vi "HFRR ADV v041.vi"() -> ()   [LabVIEW 2025] (continued)
                n816 = local write "Sample Temperature Calibration"(enum32{"True", "Fail"}."Fail" ("Sample Temperature Calibration  2")) -> ()
              }
              frame True {
                n817 = local write "Sample Temperature Calibration"(enum32{"True", "Fail"}."True" ("Sample Temperature Calibration  2")) -> ()
                n818 = property on="Accept & Save Air Temperature step 4" class="Bool (strict)"("DisabledEnum"=T19."Enabled" ("Disabled")) -> ()  [unwired: 2 in, 2 out]
              }
            }
          }
          frame #8 {
            # "CAL;END"
          }
          frame #9 {
            n819 = local write "Tab Control 4"(T12."Air Step 4" ("Tab Control 4")) -> ()
          }
        }
      }
      event "Back Stroke step main temperature": Value Change {
        n820 = event-data() -> ()  [unwired: 1 in, 6 out]
        n821 = stacked-sequence {
          frame #0 {
            n822 = Wait (ms)(milliseconds to wait=u32 1000) -> ()  [unwired: 1 out]
          }
          frame #1 {
            # "CAL;END"
            n823 = local write "Due Write"("CAL;END" ("Command")) -> ()
          }
          frame #2 {
            n824 = Wait (ms)(milliseconds to wait=u32 1000) -> ()  [unwired: 1 out]
          }
          frame #3 {
            # "CAL;END"
            n825 = local write "Due Write"("CAL;END" ("Command")) -> ()
          }
          frame #4 {
            n826 = local write "Temperature Selection"(T13."Default" ("Temperature Selection")) -> ()
            n827 = local write "Calibration Selection"(T8."Default" ("Calibration Selection")) -> ()
            n828 = local write "Main Calibration Tab"(T7."Main" ("Main Calibration Tab")) -> ()
            n829 = local write "Tab Control 4"(T12."Main" ("Tab Control 4")) -> ()
          }
        }
      }
      event "TEMPERATURE STEP  Back 4", "TEMPERATURE STEP 1 Back 3", "TEMPERATURE STEP  Back 3", "TEMPERATURE STEP 1 Back 2", "Back Air TEMPERATURE Step 4", "Back SAMPLE TEMPERATURE Step 4": Value Change {
        # "Back Stroke step main temperature"
        n830 = event-data() -> ()  [unwired: 1 in, 6 out]
        n831 = stacked-sequence {
          frame #0 {
            n832 = Wait (ms)(milliseconds to wait=u32 1000) -> ()  [unwired: 1 out]
          }
          frame #1 {
            # "CAL;END"
            n833 = local write "Due Write"("CAL;END" ("Command")) -> ()
          }
          frame #2 {
            n834 = Wait (ms)(milliseconds to wait=u32 1000) -> ()  [unwired: 1 out]
          }
          frame #3 {
            # "CAL;END"
            n835 = local write "Due Write"("CAL;END" ("Command")) -> ()
          }
          frame #4 {
            # "TEMPERATURE STEP  Back 4"
            n836 = local write "Main Calibration Tab"(T7."Temperature" ("Main Calibration Tab")) -> ()
            n837 = local write "Temperature Selection"(T13."Default" ("Temperature Selection")) -> ()
            n838 = local write "Tab Control 4"(T12."Main" ("Tab Control 4")) -> ()
            n839 = local write "Calibration Selection"(T8."Default" ("Calibration Selection")) -> ()
          }
        }
      }
      event "FF BACK", "FF BACK 2", "FF BACK 3", "FF BACK 4", "FF BACK 5", "FF BACK 6": Value Change {
        n840 = event-data() -> ()  [unwired: 1 in, 6 out]
        n841 = stacked-sequence {
          frame #0 {
            n842 = Wait (ms)(milliseconds to wait=u32 1500) -> ()  [unwired: 1 out]
          }
          frame #1 {
            n843 = local write "Due Write"("VC;0") -> ()
          }
          frame #2 {
            n844 = Wait (ms)(milliseconds to wait=u32 1500) -> ()  [unwired: 1 out]
          }
          frame #3 {
            n845 = local write "Due Write"("VC;0") -> ()
          }
          frame #4 {
            w875 = FALSE
            n846 = local write "FF BACK 2"(w875) -> ()
            n847 = local write "FF BACK 3"(w875) -> ()
            n848 = local write "FF BACK 4"(w875) -> ()
            n849 = local write "FF BACK 5"(w875) -> ()
            n850 = local write "FF BACK 6"(w875) -> ()
            n851 = local write "FF BACK"(w875) -> ()
          }
          frame #5 {
            n852 = local write "Temperature Selection"(T13."Default" ("Temperature Selection")) -> ()
            n853 = local write "Calibration Selection"(T8."Default" ("Calibration Selection")) -> ()
            n854 = local write "Friction Force Tab"(T25."Page 1" ("Friction Force Tab")) -> ()
            n855 = local write "Main Calibration Tab"(T7."Main" ("Main Calibration Tab")) -> ()
          }
        }
      }
      event "FF CONTINUE": Value Change {
        n856 = event-data() -> ()  [unwired: 1 in, 6 out]
        n857 = local write "FF CONTINUE"(FALSE ("FF CONTINUE")) -> ()
        n858 = local write "Friction Force Tab"(T25."Page 2" ("Friction Force Tab")) -> ()
      }
      event "FF CONTINUE 2": Value Change {
        n859 = event-data() -> ()  [unwired: 1 in, 6 out]
        n860 = local write "FF CONTINUE 2"(FALSE ("FF CONTINUE")) -> ()
        n861 = local write "Friction Force Tab"(T25."Page 3" ("Friction Force Tab")) -> ()
      }
      event "FF CONTINUE 3": Value Change {
        n862 = event-data() -> ()  [unwired: 1 in, 6 out]
        n863 = local write "FF CONTINUE 3"(FALSE ("FF CONTINUE")) -> ()
        n864 = local write "Friction Force Tab"(T25."Page 4" ("Friction Force Tab")) -> ()
      }
      event "FF CONTINUE 4": Value Change {
        n865 = event-data() -> ()  [unwired: 1 in, 6 out]
        n866 = local write "FF CONTINUE 4"(FALSE ("FF CONTINUE")) -> ()
        n867 = local write "Friction Force Tab"(T25."Page 5" ("Friction Force Tab")) -> ()
      }
      event "FF CONTINUE 5": Value Change {
        n868 = event-data() -> ()  [unwired: 1 in, 6 out]
        n869 = local write "FF CONTINUE 5"(FALSE ("FF CONTINUE")) -> ()
        n870 = local write "Friction Force Tab"(T25."Page 6" ("Friction Force Tab")) -> ()
      }
      event "Stroke Report Button": Value Change {
        n871 = event-data() -> ()  [unwired: 1 in, 6 out]
        n872 = local read "Point 5 - 1.0 mm"() -> (w891:bool)
        n873 = case shown="False" w891 {
          tunnel: [0.8 1.0] -> w890
          frame False {
          }
          frame True {
          }
        }
        n874 = local read "Machine Serial Number"() -> (w894:string)
        n875 = local read "USERNAME"() -> (w892:string)
        n876 = local write "Stroke Report Button"(FALSE ("Stroke Report Button")) -> ()
        n877 = call "Stroke Calibration Report.vi"("measured_value"=w890, "operator_name"=w892, "Instrument_serial Number"=w894) -> ()  [unwired: 7 in, 2 out]
      }
      event "Sample Report Button": Value Change {
        n878 = event-data() -> ()  [unwired: 1 in, 6 out]
        n879 = local read "Machine Serial Number"() -> (w900:string)
        n880 = local read "Sample 0deg temp"() -> (w897:dbl)
        n881 = local read "Sample 60deg temp"() -> (w898:dbl)
        n882 = local read "USERNAME"() -> (w899:string)
        n883 = call "Temperature Calibration Report.vi"("measured_60"=w898, "measured_zero"=w897, "operator_name"=w899, "Instrument_serial Number"=w900) -> ()  [unwired: 6 in, 2 out]
        n884 = local write "Sample Report Button"(FALSE ("Sample Report Button")) -> ()
      }
      event "Air Temperature Report Button": Value Change {
        n885 = event-data() -> ()  [unwired: 1 in, 6 out]
        n886 = local read "Machine Serial Number"() -> (w906:string)
        n887 = local read "Air 0deg temp"() -> (w903:dbl)
        n888 = local read "Air 60deg temp"() -> (w904:dbl)
        n889 = local read "USERNAME"() -> (w905:string)
        n890 = call "Air Temperature Calibration Report.vi"("measured_60"=w904, "measured_zero"=w903, "operator_name"=w905, "Instrument_serial Number"=w906) -> ()  [unwired: 6 in, 2 out]
        n891 = local write "Air Temperature Report Button"(FALSE ("Sample Report Button")) -> ()
      }
      event "Quit": Value Change {
        n892 = event-data() -> ()  [unwired: 1 in, 6 out]
      }
    }
    n893 = Wait (ms)(milliseconds to wait=u32 100) -> ()  [unwired: 1 out]
  }
  n894 = while {
    shift-right: [w909] -> _
    shift-left: "Enum - Selector" -> [w910]
    stop <- w911 stop-if-true
    # "Auto Start Logic Loop"
    n895 = case shown="\"close\"" w910 {
      tunnel: [w914 w920 w947 w979 w1009 Auto_Start_enum."Exit" ("Enum - Selector") Auto_Start_enum."Init" ("Enum - Selector")] -> w909
      frame "Init", Default {
        n896 = local read "Auto Start Test"() -> (w913:bool)
        n897 = Select(t=Auto_Start_enum."Humidity & Temperature On" ("Enum - Selector"), s=w913, f=Auto_Start_enum."Init") -> (s? t:f=w914:T15)
      }
      frame "Humidity & Temperature On" {
        n898 = stacked-sequence {
          tunnel: [_ _ _ _ _ _ Auto_Start_enum."Reach point" ("Enum - Selector")] -> w917
          frame #0 {
            w922 = T19."Disabled and Grayed Out" ("Disabled")
            w923 = TRUE ("Heater Button")
            n899 = property on="Humidity" class="Bool (strict)"("DisabledEnum"=w922) -> ()  [unwired: 2 in, 2 out]
            n900 = property on="Heater Button" class="Bool (strict)"("DisabledEnum"=w922) -> ()  [unwired: 2 in, 2 out]
            n901 = local write "Heater Button"(w923) -> ()
            n902 = local write "Humidity"(w923) -> ()
            n903 = property on="Heater Button" class="Bool (strict)"("Val(Sgnl)"=TRUE ("Value (Signaling)")) -> ()  [unwired: 2 in, 2 out]
          }
          frame #1 {
            n904 = Wait (ms)(milliseconds to wait=u32 3000) -> ()  [unwired: 1 out]
          }
          frame #2 {
            n905 = local read "Set Temp"() -> (w929:dbl)
            n906 = Number To Fractional String(number=w929, precision (6)=i16 2) -> (F-format string=w926:string)  [unwired: 2 in]
            n907 = Concatenate Strings("ST;" ("Command"), w926) -> (w927:string)
            n908 = local write "Due Write"(w927) -> ()
          }
          frame #3 {
            n909 = Wait (ms)(milliseconds to wait=u32 1500) -> ()  [unwired: 1 out]
          }
          frame #4 {
            (unwired) i16 2 ("precision (6)")
            n910 = local read "WriteHumidity"() -> (w931:string[])
            n911 = local read "Set Rh"() -> (w934:dbl)
            n912 = Number To Fractional String(number=w934) -> (F-format string=w935:string)  [unwired: 3 in]
            n913 = Concatenate Strings("M;" ("new element/subarray"), w935) -> (w936:string)
            n914 = Insert Into Array(array=w931, new element=w936) -> (w932:string[])  [unwired: 1 in]
            n915 = local write "WriteHumidity"(w932) -> ()
            n916 = local write "Due Write"("HE;1" ("Command")) -> ()
          }
          frame #5 {
            n917 = Wait (ms)(milliseconds to wait=u32 1500) -> ()  [unwired: 1 out]
          }
          frame #6 {
            w939 = TRUE ("Reach point temp")
            n918 = local write "Reach point Humidity"(w939) -> ()
            n919 = local write "Reach point temp"(w939) -> ()
          }
        }
        n920 = local read "Auto Start Test"() -> (w919:bool)
        n921 = Not(x=w919) -> (.not. x?=w918:bool)
        n922 = Select(t=Auto_Start_enum."close", s=w918, f=w917) -> (s? t:f=w920:T15)
      }
      frame "Reach point" {
        w948 = TRUE ("PAUSE")
        w956 = 1.0 ("y")
        w959 = 1.0 ("y")
        n923 = local read "Set Temp"() -> (w941:dbl)
        n924 = local read "Set Humidity:"() -> (w955:dbl)
        n925 = local read "Humidity ( %RH )"() -> (w960:dbl)
        n926 = Add(x=w941, y=w959) -> (x+y=w958:dbl)
        n927 = Subtract(x=w941, y=w959) -> (x-y=w957:dbl)
        n928 = Add(x=w955, y=w956) -> (x+y=w954:dbl)
        n929 = Subtract(x=w955, y=w956) -> (x-y=w953:dbl)
        n930 = local read "TEMP"() -> (w961:dbl)
        n931 = In Range and Coerce(upper limit=w954, x=w960, lower limit=w953) -> (In Range?=w942:bool)  [unwired: 1 out]
        n932 = In Range and Coerce(upper limit=w958, x=w961, lower limit=w957) -> (In Range?=w943:bool)  [unwired: 1 out]
        n933 = case shown="True" w942 {
          frame False {
          }
          frame True {
            n934 = case shown="True" "Reach point Humidity" {
              selector: "Reach point Humidity" -> [_ w967]
              frame False {
              }
              frame True {
                n935 = local read "EVENT LOG"() -> (w964:string)
                n936 = Not(x=w967) -> (.not. x?=w966:bool)
                n937 = local write "Reach point Humidity"(w966) -> ()
                n938 = call "Event Log.vi"("Content"="Target Humidity reached", "EVENT LOG"=w964) -> ("EVENT LOG"=w965:string)  [unwired: 8 in, 1 out]
                n939 = local write "EVENT LOG"(w965) -> ()
              }
            }
          }
        }
        n940 = case shown="True" w943 {
          frame False {
          }
          frame True {
            n941 = case shown="True" "Reach point temp" {
              selector: "Reach point temp" -> [_ w973]
              frame False {
              }
              frame True {
                n942 = local read "EVENT LOG"() -> (w970:string)
                n943 = Not(x=w973) -> (.not. x?=w972:bool)
                n944 = local write "Reach point temp"(w972) -> ()
                n945 = call "Event Log.vi"("Content"="Target Temperature reached", "EVENT LOG"=w970) -> ("EVENT LOG"=w971:string)  [unwired: 8 in, 1 out]
                n946 = local write "EVENT LOG"(w971) -> ()
              }
            }
          }
        }
        n947 = local read "Auto Start Test"() -> (w946:bool)
        n948 = And(x=w943, y=w942) -> (x .and. y?=w952:bool)
        n949 = Select(t=Auto_Start_enum."Maintain Stage" ("Enum - Selector"), s=w952, f=Auto_Start_enum."Reach point" ("Enum - Selector")) -> (s? t:f=w949:T15)
        n950 = Not(x=w946) -> (.not. x?=w945:bool)
        n951 = Select(t=Auto_Start_enum."close", s=w945, f=w949) -> (s? t:f=w947:T15)
        n952 = call "ELAPSED TIMER VI.vi"("RESET"=w948, "PAUSE"=w948) -> ()  [unwired: 7 in, 3 out]
      }
      frame "Maintain Stage" {
        w988 = 2.0 ("y")
        w987 = 1.0 ("y")
        # "Humidity and  temperatures Set Point  have been reached"
        n953 = local read "Set Temp"() -> (w974:dbl)
        n954 = local read "Set Humidity:"() -> (w991:dbl)
        n955 = local read "Humidity ( %RH )"() -> (w994:dbl)
        n956 = Add(x=w974, y=w987) -> (x+y=w993:dbl)
        n957 = Subtract(x=w974, y=w987) -> (x-y=w992:dbl)
        n958 = local read "TEMP"() -> (w995:dbl)
        n959 = Add(x=w991, y=w988) -> (x+y=w990:dbl)
        n960 = Subtract(x=w991, y=w988) -> (x-y=w989:dbl)
        n961 = In Range and Coerce(upper limit=w993, x=w995, lower limit=w992) -> (In Range?=w986:bool)  [unwired: 1 out]
        n962 = In Range and Coerce(upper limit=w990, x=w994, lower limit=w989) -> (In Range?=w985:bool)  [unwired: 1 out]
        n963 = And(x=w986, y=w985) -> (x .and. y?=w984:bool)
        n964 = Not(x=w984) -> (.not. x?=w983:bool)
        n965 = call "ELAPSED TIMER VI.vi"("TARGET"=60.0, "RESET"=w983, "PAUSE"=FALSE) -> ("ELAPSED INDICATION"=w980:bool)  [unwired: 6 in, 2 out]
        n966 = case shown="True" w980 {
          tunnel: w980 -> [_ w998]
          tunnel: [Auto_Start_enum."Maintain Stage" ("Enum - Selector") w997] -> w978
          frame False {
          }
          frame True {
            n967 = stacked-sequence {
              tunnel: w998 -> [_ _ _ _ _]
              tunnel: [_ _ _ _ Auto_Start_enum."Start Stage" ("Enum - Selector")] -> w997
              frame #0 {
                n968 = local read "EVENT LOG"() -> (w1000:string)
                n969 = call "Event Log.vi"("Content"="Humidity and temperature set point has stabilized.", "EVENT LOG"=w1000) -> ("EVENT LOG"=w1001:string)  [unwired: 8 in, 1 out]
                n970 = local write "EVENT LOG"(w1001) -> ()
              }
              frame #1 {
                n971 = Wait (ms)(milliseconds to wait=u32 100) -> ()  [unwired: 1 out]
              }
              frame #2 {
                n972 = local read "EVENT LOG"() -> (w1004:string)
                n973 = call "Event Log.vi"("Content"="Auto Test Started", "EVENT LOG"=w1004) -> ("EVENT LOG"=w1005:string)  [unwired: 8 in, 1 out]
                n974 = local write "EVENT LOG"(w1005) -> ()
              }
              frame #3 {
                w1006 = TRUE ("RUN")
                n975 = local write "RUN"(w1006) -> ()
                n976 = property on="Auto Start Temp" class="Bool (strict)"("Val(Sgnl)"=w1006) -> ()  [unwired: 2 in, 2 out]
                "Auto Start Temp" <- w1006
              }
              frame #4 {
              }
            }
          }
        }
        n977 = local read "Auto Start Test"() -> (w977:bool)
        n978 = Not(x=w977) -> (.not. x?=w976:bool)
        n979 = Select(t=Auto_Start_enum."close", s=w976, f=w978) -> (s? t:f=w979:T15)
      }
      frame "Start Stage" {
        w1008 = TRUE ("PAUSE")
        n980 = local read "Auto Start Test"() -> (w1013:bool)
        n981 = Not(x=w1013) -> (.not. x?=w1012:bool)
        n982 = Select(t=Auto_Start_enum."close" ("Enum - Selector"), s=w1012, f=Auto_Start_enum."Start Stage" ("Enum - Selector")) -> (s? t:f=w1009:T15)
        n983 = call "ELAPSED TIMER VI.vi"("RESET"=w1008, "PAUSE"=w1008) -> ()  [unwired: 7 in, 3 out]
      }
      frame "close" {
        w1016 = FALSE ("Heater Button")
        n984 = local write "RUN"(w1016) -> ()
        n985 = local write "Heater Button"(w1016) -> ()
        n986 = local write "Humidity"(w1016) -> ()
        n987 = local write "Auto Start Test"(w1016) -> ()
        n988 = property on="Heater Button" class="Bool (strict)"("Val(Sgnl)"=FALSE ("Value (Signaling)")) -> ()  [unwired: 2 in, 2 out]
        n989 = local write "Humidity 2"(TRUE ("Humidity")) -> ()
      }
      frame "Exit" {
      }
    }
    n990 = Wait (ms)(milliseconds to wait=u32 100) -> ()  [unwired: 1 out]
    n991 = local read "Quit"() -> (w911:bool)
  }
  n992 = property on="Service Password Log" class="Str"("Visible"=w23) -> ()  [unwired: 2 in, 2 out]
  n993 = property on="Password 3" class="Clust (strict)"("Visible"=w23) -> ()  [unwired: 2 in, 2 out]
  n994 = while {
    stop <- w1045 stop-if-true
    w1028 = errorcluster {"status"=FALSE, "code"=0, "source"=""} ("error in (no error) 3")
    # "this loop is for manual report generation"
    n995 = local read "Confirm Measrurement"() -> (w1027:bool)
    n996 = case shown="True" w1027 {
      selector: w1027 -> [_ w1135]
      tunnel: errorcluster {"status"=FALSE, "code"=0, "source"=""} ("error in (no error) 3") -> [_ w1136]
      tunnel: [_ w1134] -> _
      frame False {
      }
      frame True {
        n997 = stacked-sequence {
          tunnel: w1136 -> [_ w1169 _]
          tunnel: w1135 -> [_ _ w1276]
          tunnel: [_ w1157 _] -> w1134
          frame #0 {
            n998 = String To Path(string="C:\\LAB-IQ\\Image Calibrate v01.dcf") -> (path=w1139:path)
            n999 = Open/Create/Replace File ("Open File")(file path (use dialog)=w1139) -> (refnum out=w1140:refnum<file>)  [unwired: 5 in, 2 out]
            n1000 = for {
              N: 4 -> [_]
              tunnel: w1140 -> [w1146]
              i -> [w1142]
              n1001 = Read from Text File ("Read File")(file (use dialog)=w1146) -> (text=w1147:string)  [unwired: 3 in, 3 out]
              n1002 = String Subset(string=w1147, offset (0)=6, length (rest)=10 ("length (rest)")) -> (substring=w1143:string)
              n1003 = Fract/Exp String To Number(string=w1143) -> (number=w1141:dbl)  [unwired: 3 in, 1 out]
              n1004 = case shown="3" w1142 {
                tunnel: w1141 -> [w1148 w1149 _ w1150 _]
                frame 0 {
                  n1005 = local write "5x Gain"(w1148) -> ()
                }
                frame 1 {
                  n1006 = local write "10x Gain"(w1149) -> ()
                }
                frame 2 {
                }
                frame 3 {
                  n1007 = local write "100x gain"(w1150) -> ()
                }
                frame 4, Default {
                }
              }
            }
          }
          frame #1 {
            n1008 = local read "TEST STANDARD"() -> (w1152:T3)
            n1009 = case shown="\"ISO 12156\"" w1152 {
              tunnel: ["ASTM D6079" "ISO 12156"] -> w1151
              frame "ASTM D6079", Default {
              }
              frame "ISO 12156" {
              }
            }
            n1010 = call "IMAGE ANALYSIS.vi"("Enum"=POST_ANALYSIS_ENUM."GET MEASUREMENTS", "error in"=w1169) -> ("error out"=w1176:errorcluster)  [unwired: 8 in, 1 out]
            n1011 = local read "Magnification :"() -> (w1162:string)
            n1012 = call "Stall Data Flow.vim"("value in"=w1176, "milliseconds to wait"=u32 1000) -> ("value out"=w1175:errorcluster)  [unwired: 1 out]
            n1013 = local read "Test File List :"() -> (w1173:string)
            n1014 = case shown="\"10x\"" w1162 {
              tunnel: [w1212 w1213] -> w1160
              frame "5x", Default {
                n1015 = local read "5x Gain"() -> (w1212:dbl)
              }
              frame "10x" {
                # "5x"
                n1016 = local read "10x Gain"() -> (w1213:dbl)
              }
            }
            n1017 = call "IMAGE ANALYSIS.vi"("Enum"=POST_ANALYSIS_ENUM."READ", "error in"=w1175) -> ("error out"=w1172:errorcluster, "data out"=w1163:string)  [unwired: 8 in]
            n1018 = Match Pattern(string=w1163, regular expression="\"type\": ") -> (after substring=w1167:string)  [unwired: 1 in, 3 out]
            n1019 = call "IMAGE PATH CREATION PY.vi"("error in (no error)"=w1172, "File Name :"=w1173) -> ("error out"=w1171:errorcluster, "File Path"=w1159:path, "File Path String:"=w1154:string)  [unwired: 7 in]
            n1020 = Match Pattern(string=w1167, regular expression=",") -> (before substring=w1153:string)  [unwired: 1 in, 3 out]
            n1021 = local read "Calibration Tab"() -> (w1156:enum32{"Measrument", "Calibrate"})
            n1022 = call "Stall Data Flow.vim"("value in"=w1171, "milliseconds to wait"=u32 250) -> ("value out"=w1155:errorcluster)  [unwired: 1 out]
            n1023 = Equal?(x=w1153, y="\"rectangle\"") -> (x = y?=w1164:bool)
            n1024 = case shown="False" w1164 {
              tunnel: w1163 -> [w1218 w1273]
              tunnel: w1160 -> [_ w1264]
              tunnel: cluster{"major":dbl, "minor":dbl, "average":dbl} {"major"=0.0, "minor"=0.0, "average"=0.0} -> [w1216 w1260]
              tunnel: [w1215 w1257] -> w1158
              tunnel: w1153 -> [w1217 _]
              tunnel: w1160 -> [w1214 _]
              frame False {
                n1025 = Equal?(x=w1217, y="\"line\"") -> (x = y?=w1219:bool)
                n1026 = case shown="True" w1219 {
                  tunnel: w1218 -> [_ w1234]
                  tunnel: w1216 -> [w1221 w1233]
                  tunnel: [w1221 w1231] -> w1215
                  tunnel: w1214 -> [_ w1230]
                  frame False {
                  }
                  frame True {
                    w1229 = 0.0 ("Major Axis")
                    n1027 = Match Pattern(string=w1234, regular expression="\"length_px\":") -> (after substring=w1232:string)  [unwired: 1 in, 3 out]
                    n1028 = property on="Major Axis" class="DigNum (strict)"("Caption.Text"="") -> ()  [unwired: 2 in, 2 out]
                    n1029 = property on="Minor Axis" class="DigNum (strict)"("Caption.Text"="") -> ()  [unwired: 2 in, 2 out]
                    n1030 = property on="Average" class="DigNum (strict)"("Caption.Text"="Line") -> ()  [unwired: 2 in, 2 out]
                    n1031 = Fract/Exp String To Number(string=w1232, default (0 dbl)=0.0 ("default (0 DBL)")) -> (number=w1228:dbl)  [unwired: 2 in, 1 out]
                    "Pixel Value" <- w1228
                    n1032 = Multiply(x=w1228, y=w1230) -> (x*y=w1241:dbl)
                    n1033 = Multiply(x=w1241, y=1000.0) -> (x*y=w1224:dbl)
                    n1034 = Divide(x=w1224, y=1000.0) -> (x/y=w1227:dbl)
                    n1035 = local write "Measurment (mm)"(w1227) -> ()
                    n1036 = Bundle By Name(cluster=w1233, "average"=w1224) -> (w1231:cluster{"major":dbl, "minor":dbl, "average":dbl})
                    n1037 = Number To Fractional String(number=w1224, precision (6)=i16 1) -> (F-format string=w1223:string)  [unwired: 2 in]
                    n1038 = local write "Minor Axis"(w1229) -> ()
                    n1039 = local write "Major Axis"(w1229) -> ()
                    n1040 = Fract/Exp String To Number(string=w1223) -> (number=w1222:dbl)  [unwired: 3 in, 1 out]
                    n1041 = local write "Average"(w1222) -> ()
                  }
                }
              }
              frame True {
                w1261 = 1000.0 ("y")
                w1267 = 0.0 ("default (0 DBL)")
                n1042 = Match Pattern(string=w1273, regular expression=" \"width_px\":") -> (after substring=w1271:string)  [unwired: 1 in, 3 out]
                n1043 = Match Pattern(string=w1271, regular expression="\"height_px\":") -> (before substring=w1269:string, after substring=w1268:string)  [unwired: 1 in, 2 out]
                n1044 = Fract/Exp String To Number(string=w1269, default (0 dbl)=w1267) -> (number=w1266:dbl)  [unwired: 2 in, 1 out]
                n1045 = Fract/Exp String To Number(string=w1268, default (0 dbl)=w1267) -> (number=w1265:dbl)  [unwired: 2 in, 1 out]
                n1046 = Multiply(x=w1266, y=w1264) -> (x*y=w1263:dbl)
                n1047 = Multiply(x=w1265, y=w1264) -> (x*y=w1262:dbl)
                n1048 = Multiply(x=w1263, y=w1261) -> (x*y=w1247:dbl)
                n1049 = Multiply(x=w1262, y=w1261) -> (x*y=w1245:dbl)
                n1050 = Add(x=w1247, y=w1245) -> (x+y=w1259:dbl)
                n1051 = property on="Major Axis" class="DigNum (strict)"("Caption.Text"="Major Axis") -> ()  [unwired: 2 in, 2 out]
                n1052 = property on="Minor Axis" class="DigNum (strict)"("Caption.Text"="Minor Axis") -> ()  [unwired: 2 in, 2 out]
                n1053 = property on="Average" class="DigNum (strict)"("Caption.Text"="Average") -> ()  [unwired: 2 in, 2 out]
                n1054 = Divide(x=w1259, y=2.0) -> (x/y=w1243:dbl)
                n1055 = Bundle By Name(cluster=w1260, "major"=w1247, "minor"=w1245, "average"=w1243) -> (w1257:cluster{"major":dbl, "minor":dbl, "average":dbl})
                n1056 = Number To Fractional String(number=w1245, precision (6)=i16 1) -> (F-format string=w1252:string)  [unwired: 2 in]
                n1057 = Number To Fractional String(number=w1243, precision (6)=i16 1) -> (F-format string=w1253:string)  [unwired: 2 in]
                n1058 = Number To Fractional String(number=w1247, precision (6)=i16 1) -> (F-format string=w1251:string)  [unwired: 2 in]
                n1059 = Fract/Exp String To Number(string=w1252) -> (number=w1244:dbl)  [unwired: 3 in, 1 out]
                n1060 = Fract/Exp String To Number(string=w1253) -> (number=w1242:dbl)  [unwired: 3 in, 1 out]
                n1061 = Fract/Exp String To Number(string=w1251) -> (number=w1246:dbl)  [unwired: 3 in, 1 out]
                n1062 = local write "Major Axis"(w1246) -> ()
                n1063 = local write "Average"(w1242) -> ()
                n1064 = local write "Minor Axis"(w1244) -> ()
              }
            }
            n1065 = case shown="\"Measrument\", Default" w1156 {
              tunnel: w1159 -> [w1186 _]
              tunnel: w1158 -> [w1185 _]
              tunnel: [w1182 w1211] -> w1157
              tunnel: w1155 -> [w1184 w1211]
              tunnel: w1154 -> [w1183 _]
              tunnel: w1151 -> [w1181 _]
              frame "Measrument", Default {
                n1066 = stacked-sequence {
                  tunnel: w1186 -> [w1204 _]
                  tunnel: w1185 -> [w1202 _]
                  tunnel: w1184 -> [w1200 _]
                  tunnel: w1183 -> [w1199 _]
                  tunnel: [w1194 _] -> w1182
                  tunnel: w1181 -> [w1187 _]
                  frame #0 {
                    n1067 = call "IMAGE ANALYSIS.vi"("Enum"=POST_ANALYSIS_ENUM."SAVE IMAGE", "error in"=w1200, "IMAGE FILE PATH"=w1199) -> ("error out"=w1198:errorcluster)  [unwired: 7 in, 1 out]
                    n1068 = call "Stall Data Flow.vim"("value in"=w1198, "milliseconds to wait"=u32 1000) -> ("value out"=w1189:errorcluster)  [unwired: 1 out]
                    n1069 = local read "Test File List :"() -> (w1206:string)
                    n1070 = call "IMAGE ANALYSIS.vi"("Enum"=POST_ANALYSIS_ENUM."MINIMIZE UI", "error in"=w1189) -> ("error out"=w1196:errorcluster)  [unwired: 8 in, 1 out]
                    n1071 = Bundle By Name(cluster=T27 {"File Name"="", "Test Method"="", "Operator"="", "Fuel Description"="", "Date and time"=""} ("Main Ref"), "Test Method"=w1187, "File Name"=w1206) -> (w1207:T27)
                    n1072 = call "Stall Data Flow.vim"("value in"=w1196, "milliseconds to wait"=u32 1500) -> ("value out"=w1191:errorcluster)  [unwired: 1 out]
                    n1073 = call "duf file read.vi"("error in (no error)"=w1191, "Main Ref"=w1207) -> ("error out"=w1205:errorcluster, "Main Ref 2"=w1203:T27)  [unwired: 8 in]
                    n1074 = call "DETECTION REPORT for manual.vi"("error in (no error)"=w1205, "return value 3"=w1202, "Image File Path"=w1204, "Main Ref"=w1203) -> ("error out"=w1201:errorcluster)  [unwired: 7 in]
                    n1075 = call <vilib>:"Clear Errors.vi"("error in (no error)"=w1201) -> ("error out"=w1192:errorcluster)  [unwired: 5 in, 1 out]
                    n1076 = call "IMAGE ANALYSIS.vi"("Enum"=POST_ANALYSIS_ENUM."MINIMIZE UI", "error in"=w1192) -> ("error out"=w1194:errorcluster)  [unwired: 8 in, 1 out]
                  }
                  frame #1 {
                    n1077 = local write "Main Tab"(T2."HOME" ("Main Tab")) -> ()
                    n1078 = local write "Main Dashboard Buttons"(T1."Home" ("Main Dashboard Buttons")) -> ()
                  }
                }
              }
              frame "Calibrate" {
              }
            }
          }
          frame #2 {
            n1079 = Not(x=w1276) -> (.not. x?=w1275:bool)
            n1080 = local write "Confirm Measrurement"(w1275) -> ()
            n1081 = local read "Calibration Tab"() -> (w1274:enum32{"Measrument", "Calibrate"})
            n1082 = case shown="\"Measrument\", Default" w1274 {
              frame "Measrument", Default {
                (unwired) T21."HOME" ("Main Tab")
                n1083 = local write "Main Tab"(T2."HOME" ("Main Tab")) -> ()
              }
              frame "Calibrate" {
              }
            }
          }
        }
      }
    }
    n1084 = local read "Humidity"() -> (w1019:bool)
    n1085 = local read "Save Change"() -> (w1024:bool)
    n1086 = local read "Calibrate"() -> (w1025:bool)
    n1087 = local read "Auto Start Test"() -> (w1020:bool)
    n1088 = case shown="True" w1025 {
      selector: w1025 -> [_ w1132]
      frame False {
      }
      frame True {
        n1089 = Not(x=w1132) -> (.not. x?=w1131:bool)
        n1090 = local write "Calibrate"(w1131) -> ()
        n1091 = local write "Calibration Tab"(enum32{"Measrument", "Calibrate"}."Calibrate" ("Calibration Tab")) -> ()
      }
    }
    n1092 = case shown="True" w1024 {
      selector: w1024 -> [_ w1076]
      frame False {
      }
      frame True {
        n1093 = stacked-sequence {
          tunnel: w1076 -> [_ _ _ _ w1130]
          frame #0 {
            n1094 = call "IMAGE ANALYSIS.vi"("Enum"=POST_ANALYSIS_ENUM."HIDE UI") -> ()  [unwired: 9 in, 2 out]
          }
          frame #1 {
            n1095 = local read "100x gain"() -> (w1078:dbl)
            n1096 = local read "10x Gain"() -> (w1079:dbl)
            n1097 = local read "5x Gain"() -> (w1080:dbl)
            n1098 = Number To Fractional String(number=w1079, width (-)=i16 4, precision (6)=i16 7) -> (F-format string=w1101:string)  [unwired: 1 in]
            n1099 = Number To Fractional String(number=0.0, width (-)=i16 4, precision (6)=i16 7) -> (F-format string=w1096:string)  [unwired: 1 in]
            n1100 = Number To Fractional String(number=w1078, width (-)=i16 4, precision (6)=i16 7) -> (F-format string=w1084:string)  [unwired: 1 in]
            n1101 = Number To Fractional String(number=w1080, width (-)=i16 10 ("precision (6)"), precision (6)=i16 7) -> (F-format string=w1110:string)  [unwired: 1 in]
            n1102 = Concatenate Strings("[CH1]" ("string"), w1110, " - 5x Gain" ("string"), "\r") -> (w1100:string)
            n1103 = Concatenate Strings("[CH2]" ("string"), w1101, " - 10x Gain" ("string"), "\r") -> (w1099:string)
            n1104 = Concatenate Strings("[CH3]" ("string"), w1096, " - 20x Gain" ("string"), "\r") -> (w1090:string)
            n1105 = Concatenate Strings("[CH4]" ("string"), w1084, " - 100x Gain" ("string"), "\r") -> (w1083:string)
            n1106 = String To Path(string="C:\\LAB-IQ\\Image Calibrate v01.dcf") -> (path=w1113:path)
            n1107 = Concatenate Strings(w1100, w1099, w1090, w1083) -> (w1098:string)
            n1108 = call <vilib>:"Write Characters To File.vi"("append to file? (new file:F)"=FALSE, "character string"=w1098, "file path (dialog if empty)"=w1113) -> ()  [unwired: 2 in, 1 out]
          }
          frame #2 {
            n1109 = String To Path(string="C:\\LAB-IQ\\Image Calibrate v01.dcf") -> (path=w1116:path)
            n1110 = Open/Create/Replace File ("Open File")(file path (use dialog)=w1116) -> (refnum out=w1117:refnum<file>)  [unwired: 5 in, 2 out]
            n1111 = for {
              N: 4 -> [_]
              tunnel: w1117 -> [w1123]
              i -> [w1119]
              n1112 = Read from Text File ("Read File")(file (use dialog)=w1123) -> (text=w1124:string)  [unwired: 3 in, 3 out]
              n1113 = String Subset(string=w1124, offset (0)=6, length (rest)=10 ("length (rest)")) -> (substring=w1120:string)
              n1114 = Fract/Exp String To Number(string=w1120) -> (number=w1118:dbl)  [unwired: 3 in, 1 out]
              n1115 = case shown="3" w1119 {
                tunnel: w1118 -> [w1125 w1126 _ w1127 _]
                frame 0 {
                  n1116 = local write "5x Gain"(w1125) -> ()
                }
                frame 1 {
                  n1117 = local write "10x Gain"(w1126) -> ()
                }
                frame 2 {
                }
                frame 3 {
                  n1118 = local write "100x gain"(w1127) -> ()
                }
                frame 4, Default {
                }
              }
            }
          }
          frame #3 {
            n1119 = call "IMAGE ANALYSIS.vi"("Enum"=POST_ANALYSIS_ENUM."SHOW UI") -> ()  [unwired: 9 in, 2 out]
          }
          frame #4 {
            n1120 = Not(x=w1130) -> (.not. x?=w1129:bool)
            n1121 = local write "Save Change"(w1129) -> ()
          }
        }
      }
    }
    n1122 = case shown="False" w1020 {
      tunnel: w1019 -> [w1046 _]
      frame False {
        n1123 = case shown="True" w1046 {
          frame False {
          }
          frame True {
            n1124 = local read "Set Humidity:"() -> (w1050:dbl)
            n1125 = local read "Set Humidity:"() -> (w1053:dbl)
            n1126 = local read "Humidity ( %RH )"() -> (w1054:dbl)
            n1127 = Subtract(x=w1050, y=2.0) -> (x-y=w1048:dbl)
            n1128 = Add(x=w1053, y=2.0) -> (x+y=w1049:dbl)
            n1129 = In Range and Coerce(upper limit=w1049, x=w1054, lower limit=w1048) -> (In Range?=w1047:bool)  [unwired: 1 out]
            n1130 = case shown="True" w1047 {
              frame False {
              }
              frame True {
                n1131 = case shown="True" "Manual Humididty Reached" {
                  selector: "Manual Humididty Reached" -> [_ w1057]
                  frame False {
                  }
                  frame True {
                    n1132 = Not(x=w1057) -> (.not. x?=w1056:bool)
                    n1133 = local write "Manual Humididty Reached"(w1056) -> ()
                    n1134 = local read "EVENT LOG"() -> (w1059:string)
                    n1135 = call "Event Log.vi"("Content"="Target Humidity reached", "EVENT LOG"=w1059) -> ("EVENT LOG"=w1058:string)  [unwired: 8 in, 1 out]
                    n1136 = local write "EVENT LOG"(w1058) -> ()
                  }
                }
              }
            }
          }
        }
      }
      frame True {
        n1137 = local write "Manual Humididty Reached"(TRUE ("Manual Humididty Reached")) -> ()
      }
    }
    n1138 = local read "Cap Live Image"() -> (w1040:bool)
    n1139 = local read "SCAR MEASURMENT"() -> (w1043:enum32{"Auto Scar", "Manual Scar"})
    n1140 = Equal?(x=w1043, y=enum32{"Auto Scar", "Manual Scar"}."Manual Scar" ("SCAR MEASURMENT")) -> (x = y?=w1041:bool)
    n1141 = And(x=w1041, y=w1040) -> (x .and. y?=w1039:bool)
    n1142 = Wait (ms)(milliseconds to wait=u32 250) -> ()  [unwired: 1 out]
    n1143 = case shown="True" w1039 {
      selector: w1039 -> [_ w1362]
      frame False {
      }
      frame True {
        n1144 = stacked-sequence {
          tunnel: [_ _ _ w1381 _] -> _
          tunnel: w1362 -> [_ _ _ _ w1388]
          frame #0 {
            w1363 = 0.0
            n1145 = local write "Major Axis"(w1363) -> ()
            n1146 = local write "Minor Axis"(w1363) -> ()
            n1147 = local write "Average"(w1363) -> ()
          }
          frame #1 {
            n1148 = call "CAMERA LIVE FEED FGV.vi"("Enum - Menu"=CAMERA_LIVE_FEED_ENUM."CAMERA MINIMIZE") -> ()  [unwired: 9 in, 2 out]
          }
          frame #2 {
            n1149 = local read "Magnification len live scar"() -> (w1367:string)
            n1150 = case shown="\"10x\", Default" w1367 {
              tunnel: ["_10x" "_5x"] -> w1366
              frame "10x", Default {
              }
              frame "5x" {
              }
            }
            n1151 = local read "FILE 3"() -> (w1373:string)
            n1152 = call <vilib>:"Trim Whitespace.vi"("string"="C:\\LAB-IQ\\images\\") -> ("trimmed string"=w1375:string)  [unwired: 1 in]
            n1153 = String To Path(string=w1375) -> (path=w1374:path)
            n1154 = Concatenate Strings(w1373, w1366, ".png" ("string")) -> (w1372:string)
            n1155 = Build Path(base path=w1374, name or relative path=w1372) -> (appended path=w1371:path)
            n1156 = Path To String(path=w1371) -> (string=w1370:string)
            n1157 = call "CAMERA LIVE FEED FGV.vi"("Enum - Menu"=CAMERA_LIVE_FEED_ENUM."CAMERA SAVE", "Image Path"=w1370) -> ("error out"=w1368:errorcluster)  [unwired: 8 in, 1 out]
            n1158 = case shown="No Error" w1368 {
              frame No Error {
                n1159 = One Button Dialog(message="Image saved successfully") -> ()  [unwired: 1 in, 1 out]
              }
              frame Error {
              }
            }
          }
          frame #3 {
            n1160 = call "LIST FILE NAMES.vi"() -> ("error out"=w1383:errorcluster, "filenames"=w1380:string[])  [unwired: 10 in]
            n1161 = call "IMAGE ANALYSIS.vi"("Enum"=POST_ANALYSIS_ENUM."SHOW UI", "error in"=w1383) -> ("error out"=w1381:errorcluster)  [unwired: 8 in, 1 out]
            n1162 = property on="Test File List :" class="CmbBox"("Strings[]"=w1380) -> ()  [unwired: 2 in, 2 out]
          }
          frame #4 {
            (unwired) T26."Report" ("Main Dashboard Buttons")
            (unwired) T28."Report" ("Main Dashboard Buttons")
            n1163 = Not(x=w1388) -> (.not. x?=w1387:bool)
            n1164 = local write "Zoom Factore"(0.0 ("Zoom Factore")) -> ()
            n1165 = local write "Cap Live Image"(w1387) -> ()
            n1166 = local write "Main Tab"(T2."Adv Scar Report" ("Main Tab")) -> ()
            n1167 = property on="Cap Live Image" class="Bool (strict)"("BoolText.Text"="Capture Image" ("Boolean Text.Text")) -> ()  [unwired: 2 in, 2 out]
            n1168 = local write "Main Dashboard Buttons"(T1."Report" ("Main Dashboard Buttons")) -> ()
          }
        }
      }
    }
    n1169 = local read "change Gain"() -> (w1023:bool)
    n1170 = local read "Back Square"() -> (w1022:bool)
    n1171 = case shown="True" w1023 {
      selector: w1023 -> [_ w1067]
      frame False {
      }
      frame True {
        n1172 = stacked-sequence {
          tunnel: w1067 -> [_ w1075]
          frame #0 {
            n1173 = local read "Actual (µm)"() -> (w1071:dbl)
            n1174 = local read "Pixel Value"() -> (w1070:dbl)
            n1175 = local read "Magnification :"() -> (w1069:string)
            n1176 = Divide(x=w1071, y=w1070) -> (x/y=w1068:dbl)
            n1177 = case shown="\"10x\"" w1069 {
              tunnel: w1068 -> [w1072 w1073]
              frame "10x" {
                n1178 = local write "10x Gain"(w1072) -> ()
              }
              frame "5x", Default {
                n1179 = local write "5x Gain"(w1073) -> ()
              }
            }
          }
          frame #1 {
            n1180 = Not(x=w1075) -> (.not. x?=w1074:bool)
            n1181 = local write "change Gain"(w1074) -> ()
          }
        }
      }
    }
    n1182 = case shown="True" w1022 {
      selector: w1022 -> [_ w1065]
      frame False {
      }
      frame True {
        n1183 = Not(x=w1065) -> (.not. x?=w1064:bool)
        n1184 = local write "Back Square"(w1064) -> ()
        n1185 = local write "Calibration Tab"(enum32{"Measrument", "Calibrate"}."Measrument" ("Calibration Tab")) -> ()
      }
    }
    n1186 = local read "Rectangle Tool"() -> (w1034:bool)
    n1187 = local read "Clear ROI Tool"() -> (w1033:bool)
    n1188 = local read "Open Image"() -> (w1038:bool)
    n1189 = local read "line tool"() -> (w1035:bool)
    n1190 = local read "OUT"() -> (w1036:bool)
    n1191 = local read "In"() -> (w1037:bool)
    n1192 = case shown="True" w1038 {
      selector: w1038 -> [_ w1348]
      tunnel: [w1339 w1350] -> _
      tunnel: w1028 -> [w1339 w1349]
      frame False {
      }
      frame True {
        w1343 = "_5x" ("regular expression")
        n1193 = Not(x=w1348) -> (.not. x?=w1347:bool)
        n1194 = local write "Open Image"(w1347) -> ()
        n1195 = call "IMAGE ANALYSIS.vi"("Enum"=POST_ANALYSIS_ENUM."HIDE UI", "error in"=w1349) -> ("error out"=w1357:errorcluster)  [unwired: 8 in, 1 out]
        n1196 = call <vilib>:"Clear Errors.vi"("error in (no error)"=w1357) -> ("error out"=w1340:errorcluster)  [unwired: 5 in, 1 out]
        n1197 = call "File Dialog"("start path"=path "C:/LAB-IQ/images", "error in"=w1340) -> ("selected path"=w1342:path, "error out"=w1355:errorcluster)  [unwired: 10 in, 2 out]
        "Image path  2" <- w1342
        n1198 = call <vilib>:"Clear Errors.vi"("error in (no error)"=w1355) -> ("error out"=w1354:errorcluster)  [unwired: 5 in, 1 out]
        n1199 = call "IMAGE ANALYSIS.vi"("Enum"=POST_ANALYSIS_ENUM."OPEN FILE", "error in"=w1354, "File Path"=w1342) -> ("error out"=w1353:errorcluster)  [unwired: 7 in, 1 out]
        n1200 = call <vilib>:"Clear Errors.vi"("error in (no error)"=w1353) -> ("error out"=w1352:errorcluster)  [unwired: 5 in, 1 out]
        n1201 = call "IMAGE ANALYSIS.vi"("Enum"=POST_ANALYSIS_ENUM."SHOW UI", "error in"=w1352) -> ("error out"=w1350:errorcluster)  [unwired: 8 in, 1 out]
        n1202 = local write "Zoom Factore"(100.0 ("Zoom Factore")) -> ()
        n1203 = Strip Path(path=w1342) -> (name=w1345:string)  [unwired: 1 out]
        n1204 = Match Pattern(string=w1345, regular expression=w1343) -> (match substring=w1344:string)  [unwired: 1 in, 3 out]
        n1205 = Equal?(x=w1344, y=w1343) -> (x = y?=w1341:bool)
        n1206 = case shown="False" w1341 {
          frame False {
            n1207 = local write "Magnification :"("10x" ("Magnification :")) -> ()
          }
          frame True {
            n1208 = local write "Magnification :"("5x" ("Magnification :")) -> ()
          }
        }
      }
    }
    n1209 = case shown="True" w1036 {
      selector: w1036 -> [_ w1324]
      tunnel: w1028 -> [w1321 w1329]
      tunnel: [w1321 w1323] -> _
      frame False {
      }
      frame True {
        n1210 = Not(x=w1324) -> (.not. x?=w1322:bool)
        n1211 = local read "Zoom Factore"() -> (w1327:dbl)
        n1212 = local write "OUT"(w1322) -> ()
        n1213 = call "IMAGE ANALYSIS.vi"("Enum"=POST_ANALYSIS_ENUM."ZOOM OUT", "error in"=w1329) -> ("error out"=w1323:errorcluster)  [unwired: 8 in, 1 out]
        n1214 = Divide(x=w1327, y=1.2) -> (x/y=w1325:dbl)
        n1215 = local write "Zoom Factore"(w1325) -> ()
      }
    }
    n1216 = case shown="True" w1037 {
      selector: w1037 -> [_ w1333]
      tunnel: w1028 -> [w1330 w1338]
      tunnel: [w1330 w1331] -> _
      frame False {
      }
      frame True {
        n1217 = Not(x=w1333) -> (.not. x?=w1332:bool)
        n1218 = local read "Zoom Factore"() -> (w1336:dbl)
        n1219 = local write "In"(w1332) -> ()
        n1220 = call "IMAGE ANALYSIS.vi"("Enum"=POST_ANALYSIS_ENUM."ZOOM IN", "error in"=w1338) -> ("error out"=w1331:errorcluster)  [unwired: 8 in, 1 out]
        n1221 = Multiply(x=w1336, y=1.2) -> (x*y=w1334:dbl)
        n1222 = local write "Zoom Factore"(w1334) -> ()
      }
    }
    n1223 = case shown="True" w1033 {
      selector: w1033 -> [_ w1305]
      tunnel: w1028 -> [w1303 w1307]
      tunnel: [w1303 w1306] -> _
      frame False {
      }
      frame True {
        n1224 = Not(x=w1305) -> (.not. x?=w1304:bool)
        n1225 = local write "Clear ROI Tool"(w1304) -> ()
        n1226 = call "IMAGE ANALYSIS.vi"("Enum"=POST_ANALYSIS_ENUM."CLEAR ROI", "error in"=w1307) -> ("error out"=w1306:errorcluster)  [unwired: 8 in, 1 out]
      }
    }
    n1227 = case shown="True" w1035 {
      selector: w1035 -> [_ w1317]
      tunnel: w1028 -> [w1315 w1320]
      tunnel: [w1315 w1318] -> _
      frame False {
      }
      frame True {
        n1228 = Not(x=w1317) -> (.not. x?=w1316:bool)
        n1229 = local write "line tool"(w1316) -> ()
        n1230 = call "IMAGE ANALYSIS.vi"("Enum"=POST_ANALYSIS_ENUM."DRAW LINE", "error in"=w1320) -> ("error out"=w1318:errorcluster)  [unwired: 8 in, 1 out]
      }
    }
    n1231 = case shown="True" w1034 {
      selector: w1034 -> [_ w1311]
      tunnel: w1028 -> [w1309 w1313]
      tunnel: [w1309 w1312] -> _
      frame False {
      }
      frame True {
        n1232 = Not(x=w1311) -> (.not. x?=w1310:bool)
        n1233 = local write "Rectangle Tool"(w1310) -> ()
        n1234 = call "IMAGE ANALYSIS.vi"("Enum"=POST_ANALYSIS_ENUM."DRAW REC", "error in"=w1313) -> ("error out"=w1312:errorcluster)  [unwired: 8 in, 1 out]
      }
    }
    n1235 = local read "SCAR MEASURMENT"() -> (w1021:enum32{"Auto Scar", "Manual Scar"})
    n1236 = local read "Fit to Screen Tool"() -> (w1030:bool)
    n1237 = local read "Resize Tool"() -> (w1029:bool)
    n1238 = case shown="\"Manual Scar\", Default" w1021 {
      frame "Auto Scar" {
        n1239 = property on="Cap Live Image" class="Bool (strict)"("BoolText.Text"="Report" ("Boolean Text.Text")) -> ()  [unwired: 2 in, 2 out]
      }
      frame "Manual Scar", Default {
        n1240 = property on="Cap Live Image" class="Bool (strict)"("BoolText.Text"="Save Image" ("Boolean Text.Text")) -> ()  [unwired: 2 in, 2 out]
      }
    }
    n1241 = local read "ROI Color Tool"() -> (w1031:bool)
    n1242 = local read "Pan Tool"() -> (w1032:bool)
    n1243 = case shown="True" w1032 {
      selector: w1032 -> [_ w1299]
      tunnel: w1028 -> [w1297 w1301]
      tunnel: [w1297 w1300] -> _
      frame False {
      }
      frame True {
        n1244 = Not(x=w1299) -> (.not. x?=w1298:bool)
        n1245 = call "IMAGE ANALYSIS.vi"("Enum"=POST_ANALYSIS_ENUM."PAN", "error in"=w1301) -> ("error out"=w1300:errorcluster)  [unwired: 8 in, 1 out]
        n1246 = local write "Pan Tool"(w1298) -> ()
      }
    }
    n1247 = case shown="True" w1029 {
      selector: w1029 -> [_ w1283]
      tunnel: w1028 -> [w1278 w1280]
      tunnel: [w1278 w1279] -> _
      frame False {
      }
      frame True {
        n1248 = Not(x=w1283) -> (.not. x?=w1282:bool)
        n1249 = local write "Resize Tool"(w1282) -> ()
        n1250 = call "IMAGE ANALYSIS.vi"("Enum"=POST_ANALYSIS_ENUM."RESIZE MODE", "error in"=w1280) -> ("error out"=w1279:errorcluster)  [unwired: 8 in, 1 out]
      }
    }
    n1251 = case shown="True" w1030 {
      selector: w1030 -> [_ w1288]
      tunnel: [w1284 w1289] -> _
      tunnel: w1028 -> [w1284 w1287]
      frame False {
      }
      frame True {
        n1252 = Not(x=w1288) -> (.not. x?=w1286:bool)
        n1253 = local write "Zoom Factore"(100.0 ("Zoom Factore")) -> ()
        n1254 = local write "Fit to Screen Tool"(w1286) -> ()
        n1255 = call "IMAGE ANALYSIS.vi"("Enum"=POST_ANALYSIS_ENUM."FIT", "error in"=w1287) -> ("error out"=w1289:errorcluster)  [unwired: 8 in, 1 out]
      }
    }
    n1256 = case shown="True" w1031 {
      selector: w1031 -> [_ w1294]
      tunnel: [w1291 w1295] -> _
      tunnel: w1028 -> [w1291 w1292]
      frame False {
      }
      frame True {
        n1257 = Not(x=w1294) -> (.not. x?=w1293:bool)
        n1258 = local write "ROI Color Tool"(w1293) -> ()
        n1259 = call "IMAGE ANALYSIS.vi"("Enum"=POST_ANALYSIS_ENUM."SET ROI COLOR", "error in"=w1292) -> ("error out"=w1295:errorcluster)  [unwired: 8 in, 1 out]
      }
    }
    n1260 = local read "Quit"() -> (w1045:bool)
  }
  n1261 = while {
    stop <- w1390 stop-if-true
    n1262 = local read "Image Path"() -> (w1393:path)
    n1263 = local read "Print 3"() -> (w1396:bool)
    n1264 = Equal?(x=w1393, y=path "") -> (x = y?=w1392:bool)
    n1265 = Not(x=w1392) -> (.not. x?=w1391:bool)
    n1266 = property on="Print 3" class="Bool (strict)"("Visible"=w1391) -> ()  [unwired: 2 in, 2 out]
    n1267 = case shown="True" w1396 {
      frame False {
        n1268 = local write "Rd"(TRUE ("Boolean 7")) -> ()
      }
      frame True {
        n1269 = flat-sequence {
          tunnel: [w1436] -> w1404
          tunnel: [w1423] -> w1402
          tunnel: [w1433] -> w1398
          tunnel: w1404 -> [w1445]
          tunnel: [w1445] -> w1403
          tunnel: w1402 -> [w1444]
          tunnel: [w1444] -> w1401
          tunnel: [w1442] -> w1400
          tunnel: [w1441] -> w1399
          tunnel: w1398 -> [w1441]
          tunnel: w1403 -> [w1447]
          tunnel: w1401 -> [w1448]
          tunnel: w1400 -> [_]
          tunnel: w1399 -> [w1446]
          frame #0 {
            n1270 = case shown="True" "Rd" {
              frame False {
              }
              frame True {
                n1271 = while {
                  tunnel: "abcdefABCDEF" ("string 2") -> [w1415]
                  shift-right: [w1413] -> w1407
                  shift-left: "" -> [w1412]
                  i -> [w1422]
                  stop <- w1421 stop-if-true
                  n1272 = Random Number (0-1)() -> (number: 0 to 1=w1416:dbl)
                  n1273 = Multiply(x=w1416, y=62.0) -> (x*y=w1418:dbl)
                  n1274 = Decrement(x="Length 2") -> (x-1=w1411:i16)
                  n1275 = To Word Integer(number=w1418) -> (16bit integer=w1419:i16)
                  n1276 = String Subset(string=w1415, offset (0)=w1419, length (rest)=1 ("length (rest)")) -> (substring=w1414:string)
                  n1277 = Greater Or Equal?(x=w1422, y=w1411) -> (x >= y?=w1421:bool)
                  n1278 = Concatenate Strings(w1414, w1412) -> (w1413:string)
                }
                "String 10" <- w1407
                n1279 = local write "Rd"(FALSE ("Boolean 7")) -> ()
              }
            }
          }
          frame #1 {
            w1434 = "_resized.jpg" ("command line")
            (unwired) ".jpg -resize 320x240 " ("string")
            (unwired) "Choose an Image File" ("prompt")
            # "-resize 1798x425"
            n1280 = local read "Image Path"() -> (w1428:path)
            n1281 = Strip Path(path=w1428) -> (stripped path=w1423:path, name=w1424:string)
            n1282 = Match Pattern(string=w1424, regular expression=".jpg") -> (before substring=→"before substring 2":string, after substring=→"after substring":string)  [unwired: 1 in, 2 out]
            n1283 = Match Pattern(string=w1424, regular expression="\\") -> (before substring=w1430:string)  [unwired: 1 in, 3 out]
            n1284 = Match Pattern(string=w1430, regular expression=".jpg") -> (before substring=w1429:string)  [unwired: 1 in, 3 out]
            n1285 = Concatenate Strings("cmd /c convert " ("string"), w1429, ".jpg -resize 320x240  " ("command line"), w1429, w1434) -> (w1437:string)
            n1286 = call <vilib>:"System Exec.vi"("run minimized? (F)"=TRUE, "wait until completion? (T)"=TRUE, "working directory"=w1423, "command line"=w1437) -> ("error out"=w1436:errorcluster)  [unwired: 4 in, 3 out]
            "error out 2" <- w1436
            n1287 = Concatenate Strings(w1429, w1434) -> (w1433:string)
          }
          frame #2 {
            n1288 = Wait (ms)(milliseconds to wait=u32 2000 ("millisecond timer value")) -> (millisecond timer value=w1442:u32)
          }
          frame #3 {
            n1289 = case shown="No Error" w1447 {
              tunnel: w1448 -> [w1451 _]
              tunnel: w1446 -> [w1449 _]
              frame No Error {
                (unwired) ".jpg" ("string")
                n1290 = Path To String(path=w1451) -> (string=w1455:string)
                n1291 = Concatenate Strings(w1455, "\\" ("string"), w1449) -> (w1454:string)
                n1292 = String To Path(string=w1454) -> (path=w1453:path)
                n1293 = call <vilib>:"Read JPEG File.vi"("path to JPEG file"=w1453) -> ("image data"=w1457:T16)  [unwired: 8 in, 2 out]
                "image data" <- w1457
                n1294 = local write "Print 3"(FALSE ("Print 2")) -> ()
                n1295 = call <vilib>:"Draw Flattened Pixmap.vi"("image data"=w1457) -> ("new picture"=→"new picture":picture)  [unwired: 8 in]
              }
              frame Error {
              }
            }
          }
        }
      }
    }
    n1296 = Wait (ms)(milliseconds to wait=u32 20 ("millisecond timer value")) -> ()  [unwired: 1 out]
    n1297 = local read "Quit"() -> (w1390:bool)
  }
  n1298 = while {
    tunnel: w40 -> [_]
    tunnel: w26 -> [_]
    stop <- w1487 stop-if-true
    # "New Adv Logics"
    n1299 = local read "Main Tab"() -> (w1468:T2)
    n1300 = local read "Main Tab"() -> (w1485:T2)
    n1301 = local read "Sign In"() -> (w1484:bool)
    n1302 = case shown="\"Adv Scar\"" w1468 {
      frame "HOME", Default {
        n1303 = local read "LIVE FEED MIN TEMP"() -> (w1620:bool)
        n1304 = local write "LIVE FEED MAX TEMP"(TRUE ("LIVE FEED MAX TEMP")) -> ()
        n1305 = local read "CAMERA ROI MIN TEMP"() -> (w1618:bool)
        n1306 = case shown="True" w1620 {
          selector: w1620 -> [_ w1627]
          frame False {
          }
          frame True {
            n1307 = Not(x=w1627) -> (.not. x?=w1626:bool)
            n1308 = local write "LIVE FEED MIN TEMP"(w1626) -> ()
            n1309 = call "CAMERA LIVE FEED FGV.vi"("Enum - Menu"=CAMERA_LIVE_FEED_ENUM."CAMERA MINIMIZE") -> ()  [unwired: 9 in, 2 out]
          }
        }
        n1310 = case shown="True" w1618 {
          selector: w1618 -> [_ w1624]
          frame False {
          }
          frame True {
            n1311 = Not(x=w1624) -> (.not. x?=w1623:bool)
            n1312 = local write "CAMERA ROI MIN TEMP"(w1623) -> ()
            n1313 = call "IMAGE ANALYSIS.vi"("Enum"=POST_ANALYSIS_ENUM."MINIMIZE UI") -> ()  [unwired: 9 in, 2 out]
          }
        }
        n1314 = local write "CAMERA ROI MAX TEMP"(TRUE ("CAMERA ROI MAX TEMP")) -> ()
      }
      frame "Test Setup" {
        n1315 = local read "LIVE FEED MIN TEMP"() -> (w1630:bool)
        n1316 = local read "CAMERA ROI MIN TEMP"() -> (w1628:bool)
        n1317 = local write "LIVE FEED MAX TEMP"(TRUE ("LIVE FEED MAX TEMP")) -> ()
        n1318 = case shown="True" w1630 {
          selector: w1630 -> [_ w1637]
          frame False {
          }
          frame True {
            n1319 = Not(x=w1637) -> (.not. x?=w1636:bool)
            n1320 = local write "LIVE FEED MIN TEMP"(w1636) -> ()
            n1321 = call "CAMERA LIVE FEED FGV.vi"("Enum - Menu"=CAMERA_LIVE_FEED_ENUM."CAMERA MINIMIZE") -> ()  [unwired: 9 in, 2 out]
          }
        }
        n1322 = case shown="True" w1628 {
          selector: w1628 -> [_ w1634]
          frame False {
          }
          frame True {
            n1323 = Not(x=w1634) -> (.not. x?=w1633:bool)
            n1324 = local write "CAMERA ROI MIN TEMP"(w1633) -> ()
            n1325 = call "IMAGE ANALYSIS.vi"("Enum"=POST_ANALYSIS_ENUM."MINIMIZE UI") -> ()  [unwired: 9 in, 2 out]
          }
        }
        n1326 = local write "CAMERA ROI MAX TEMP"(TRUE ("CAMERA ROI MAX TEMP")) -> ()
      }
      frame "Acquire" {
        n1327 = local read "LIVE FEED MIN TEMP"() -> (w1640:bool)
        n1328 = local write "LIVE FEED MAX TEMP"(TRUE ("LIVE FEED MAX TEMP")) -> ()
        n1329 = local read "CAMERA ROI MIN TEMP"() -> (w1638:bool)
        n1330 = case shown="True" w1640 {
          selector: w1640 -> [_ w1647]
          frame False {
          }
          frame True {
            n1331 = Not(x=w1647) -> (.not. x?=w1646:bool)
            n1332 = local write "LIVE FEED MIN TEMP"(w1646) -> ()
            n1333 = call "CAMERA LIVE FEED FGV.vi"("Enum - Menu"=CAMERA_LIVE_FEED_ENUM."CAMERA MINIMIZE") -> ()  [unwired: 9 in, 2 out]
          }
        }
        n1334 = case shown="True" w1638 {
          selector: w1638 -> [_ w1644]
          frame False {
          }
          frame True {
            n1335 = Not(x=w1644) -> (.not. x?=w1643:bool)
            n1336 = local write "CAMERA ROI MIN TEMP"(w1643) -> ()
            n1337 = call "IMAGE ANALYSIS.vi"("Enum"=POST_ANALYSIS_ENUM."MINIMIZE UI") -> ()  [unwired: 9 in, 2 out]